vi "HeartBeatDetectOffline2Valsalva.vi"() -> ()   [LabVIEW 2014, in "Phonocardiography.lvlib"]
uses:
  Phonocardiography.lvlib
  <vilib>/Waveform/WDTOps.llb/WDT Index Channel DBL.vi
  <vilib>/Waveform/WDTOps.llb/WDT Get Waveform Time Array DBL.vi
  <vilib>/gmath/NI_Gmath.lvlib
  <vilib>/Analysis/NI_AALBase.lvlib
panel:
  in  "Exhale Length [s]":dbl=20.0
  out "RR intervals Spectra":T1(graph)={"Power Spectrum FFT {X} Frequency"=[0.0, 0.025494335748261657, 0.050988671496523315, 0.07648300724478498, 0.10197734299304663, 0.1274716787413083, 0.15296601448956995, 0.1784603502378316, 0.20395468598609326, 0.2294490217343549, 0.2549433574826166, 0.28043769323087825, 0.3059320289791399, 0.33142636472740156, 0.3569207004756632, 0.38241503622392486, 0.4079093719721865, 0.4334037077204482, 0.4588980434687098, 0.4843923792169715, 0.5098867149652332, 0.5353810507134948, 0.5608753864617565, 0.5863697222100182, 0.6118640579582798, 0.6373583937065415, 0.6628527294548031, 0.6883470652030648, 0.7138414009513264, 0.7393357366995881, 0.7648300724478497, 0.7903244081961114, 0.815818743944373, 0.8413130796926347, 0.8668074154408963, 0.892301751189158, 0.9177960869374197, 0.9432904226856813, 0.968784758433943, 0.9942790941822046, 1.0197734299304664, 1.045267765678728, 1.0707621014269897, 1.0962564371752512, 1.121750772923513, 1.1472451086717745, 1.1727394444200363, 1.1982337801682978, 1.2237281159165596, 1.2492224516648212, 1.274716787413083, 1.3002111231613445, 1.3257054589096062, 1.3511997946578678, 1.3766941304061295, 1.402188466154391, 1.4276828019026528, 1.4531771376509144, 1.4786714733991762], "Power Spectrum FFT {X}"=[6.194748647147158e-24, 9229.548494920025, 1188.4920860052935, 947.8842969704942, 178.63197208555547, 71.46762690308067, 205.39345276047945, 144.27075798793635, 81.13456035019907, 14.233100403863002, 70.63257760443297, 81.86763326737034, 31.359253750538112, 38.78063411373954, 63.199253406710866, 37.96608881281612, 1.8581095317295782, 7.247275056105265, 3.888477791210256, 19.078038441682054, 43.408583710979855, 31.794851712590184, 23.507910464090752, 3.0603332942735766, 9.734464709591705, 7.800318484915491, 22.688612828789623, 46.34799950953906, 30.540582735785772, 17.053473818925937, 5.267363301568957, 26.95792599083291, 10.575021658989519, 26.04160962099042, 119.40238100275175, 39.36493765074656, 47.92746655778191, 26.235986845520635, 199.6106688709268, 677.5407288058668, 356.86867414086265, 1572.0901514152968, 2451.586051527142, 477.6196783700457, 610.6344556635514, 1181.337476994924, 128.33756322878241, 687.9177159050421, 1078.297501063014, 1180.2511971323859, 289.91558302839945, 85.34770217036714, 78.25445989986403, 7.873565805919232, 82.9457034917068, 122.5040965317584, 14.428981027927678, 14.60917219116577, 2.0649497624039586]}
  in  "Remove\nEctopic Beats":bool=TRUE
  out "pNN50 [%]":dbl=10.344827586206897 format="%.1f"
  out "rMSSD  [ms] 2":dbl=56.69079988743271
  out "sdRR [ms]":dbl=155.73913956064249
  out "Mean RR [ms]":dbl=679.0314769975785 format="%_1f"
  out "Mean heart rate [BPM]":dbl=88.36114676936246 format="%#.1g"
  in  "Negate":bool
  out "Heart rate":T2(graph)=[{"X [s]"=[0.9536507936507932, 1.7804988662131511, 2.524807256235827, 3.2744671201814044, 4.085170068027209, 4.935691609977322, 5.717823129251698, 6.664217687074827, 7.49442176870748, 8.24662131519274, 8.931065759637184, 9.6128798185941, 10.405986394557818, 11.348027210884348, 12.258866213151922, 13.136780045351468, 13.961088435374144, 14.727165532879813, 15.434376417233553, 16.08961451247165, 16.721904761904756, 17.338321995464845, 17.933514739229018, 18.513469387755094, 19.077641723356003, 19.63292517006802, 20.182403628117907, 20.724172335600898, 21.26467120181405, 21.80018140589568, 22.325532879818585, 22.852698412698402, 23.38702947845804, 23.93859410430838, 24.48843537414965, 25.032743764172324, 25.566167800453503, 26.094965986394545, 26.626666666666654, 27.148843537414955, 27.667120181405885, 28.183219954648514, 28.69315192743763, 29.19600907029477, 29.70113378684806, 30.20426303854874, 30.718911564625838, 31.25142857142856, 31.85287981859409, 32.489795918367335, 33.11401360544216, 33.734331065759626, 34.587845804988646, 35.485986394557806, 36.427664399092954, 37.37106575963717, 38.321088435374136, 39.26984126984125, 40.178049886621295], "Heart Rate [BPM]"=[71.55993076590225, 72.56472136902153, 80.61174750182794, 80.03629764065343, 74.00984560304319, 70.54495041057912, 76.71344079786621, 63.39850488786662, 72.27138643067849, 79.76606776799711, 87.66233766233783, 88.0005321271783, 75.65187557182081, 63.69150779896015, 65.87333200557657, 68.34383717326173, 72.78829225352112, 78.32109874496807, 84.84032320123139, 91.56976744186045, 94.89312867594295, 97.33666862860537, 100.80768058518736, 103.45636534250875, 106.35048231511234, 108.05292388108468, 109.19445361505448, 110.74836765444552, 111.00855848296688, 112.04268292682941, 114.20925414364623, 113.81624225739887, 112.28993379731786, 108.78145041933905, 109.12240184757502, 110.2316280619899, 112.48087060023806, 113.4648370497429, 112.84544524053209, 114.90359562271999, 115.76828841442064, 116.25659050966627, 117.6627534685167, 119.31818181818207, 118.78254623810332, 119.25365062195846, 116.58442016214268, 112.67245784363834, 99.75870909365125, 94.20393050412952, 96.12031386225006, 96.72466734902676, 70.29755579171136, 66.80468592203607, 63.716047004430656, 63.599653879434875, 63.15638724460529, 63.240917782027125, 66.06411664835723]}, {"X [s]"=array[450560 elements], "Heart Rate [BPM]"=array[450560 elements]}]
  out "Heart beats":cluster{"Peaks X":dbl[], "Peaks Y":dbl[]}[](graph)=[{"Peaks X"=array[450560 elements], "Peaks Y"=array[450560 elements]}, {"Peaks X"=[0.11519274376417228, 0.9536507936507932, 1.7804988662131511, 2.524807256235827, 3.2744671201814044, 4.085170068027209, 4.935691609977322, 5.717823129251698, 6.664217687074827, 7.49442176870748, 8.24662131519274, 8.931065759637184, 9.6128798185941, 10.405986394557818, 11.348027210884348, 12.258866213151922, 13.136780045351468, 13.961088435374144, 14.727165532879813, 15.434376417233553, 16.08961451247165, 16.721904761904756, 17.338321995464845, 17.933514739229018, 18.513469387755094, 19.077641723356003, 19.63292517006802, 20.182403628117907, 20.724172335600898, 21.26467120181405, 21.80018140589568, 22.325532879818585, 22.852698412698402, 23.38702947845804, 23.93859410430838, 24.48843537414965, 25.032743764172324, 25.566167800453503, 26.094965986394545, 26.626666666666654, 27.148843537414955, 27.667120181405885, 28.183219954648514, 28.69315192743763, 29.19600907029477, 29.70113378684806, 30.20426303854874, 30.718911564625838, 31.25142857142856, 31.85287981859409, 32.489795918367335, 33.11401360544216, 33.734331065759626, 34.587845804988646, 35.485986394557806, 36.427664399092954, 37.37106575963717, 38.321088435374136, 39.26984126984125, 40.178049886621295], "Peaks Y"=[0.26409912109375, 0.216064453125, 0.231689453125, 0.2972412109375, 0.2186279296875, 0.310516357421875, 0.252410888671875, 0.3045654296875, 0.187164306640625, 0.24078369140625, 0.215057373046875, 0.3526611328125, 0.2615966796875, 0.229461669921875, 0.192779541015625, 0.189361572265625, 0.17205810546875, 0.186737060546875, 0.212005615234375, 0.185272216796875, 0.16400146484375, 0.175933837890625, 0.1873779296875, 0.1800537109375, 0.20709228515625, 0.20452880859375, 0.2001953125, 0.218231201171875, 0.222015380859375, 0.217681884765625, 0.201202392578125, 0.212066650390625, 0.219879150390625, 0.2449951171875, 0.2816162109375, 0.262664794921875, 0.234039306640625, 0.287567138671875, 0.267730712890625, 0.258544921875, 0.271209716796875, 0.25408935546875, 0.272186279296875, 0.230987548828125, 0.265380859375, 0.269317626953125, 0.267486572265625, 0.289703369140625, 0.216644287109375, 0.20257568359375, 0.270477294921875, 0.246978759765625, 0.403839111328125, 0.436309814453125, 0.427947998046875, 0.40887451171875, 0.40252685546875, 0.448974609375, 0.42376708984375, 0.371551513671875]}]
  in  "Max time to peak\nfrom threshold (ms)":dbl=150.0
  in  "Threshold mult 2":dbl=0.35 min=-1.0 max=1.0 step=0.05
  in  "Min time between\nbeats (ms)":dbl=400.0
  in  "width (threshold) 2":i32=3
  in  "File Path Control":path=path "C:/Users/Tamas/Documents/Projektek/Magzati szívhang/Felvételek cikkhez/valsalva5.wav"
  in  "Init length [s]":dbl=10.0
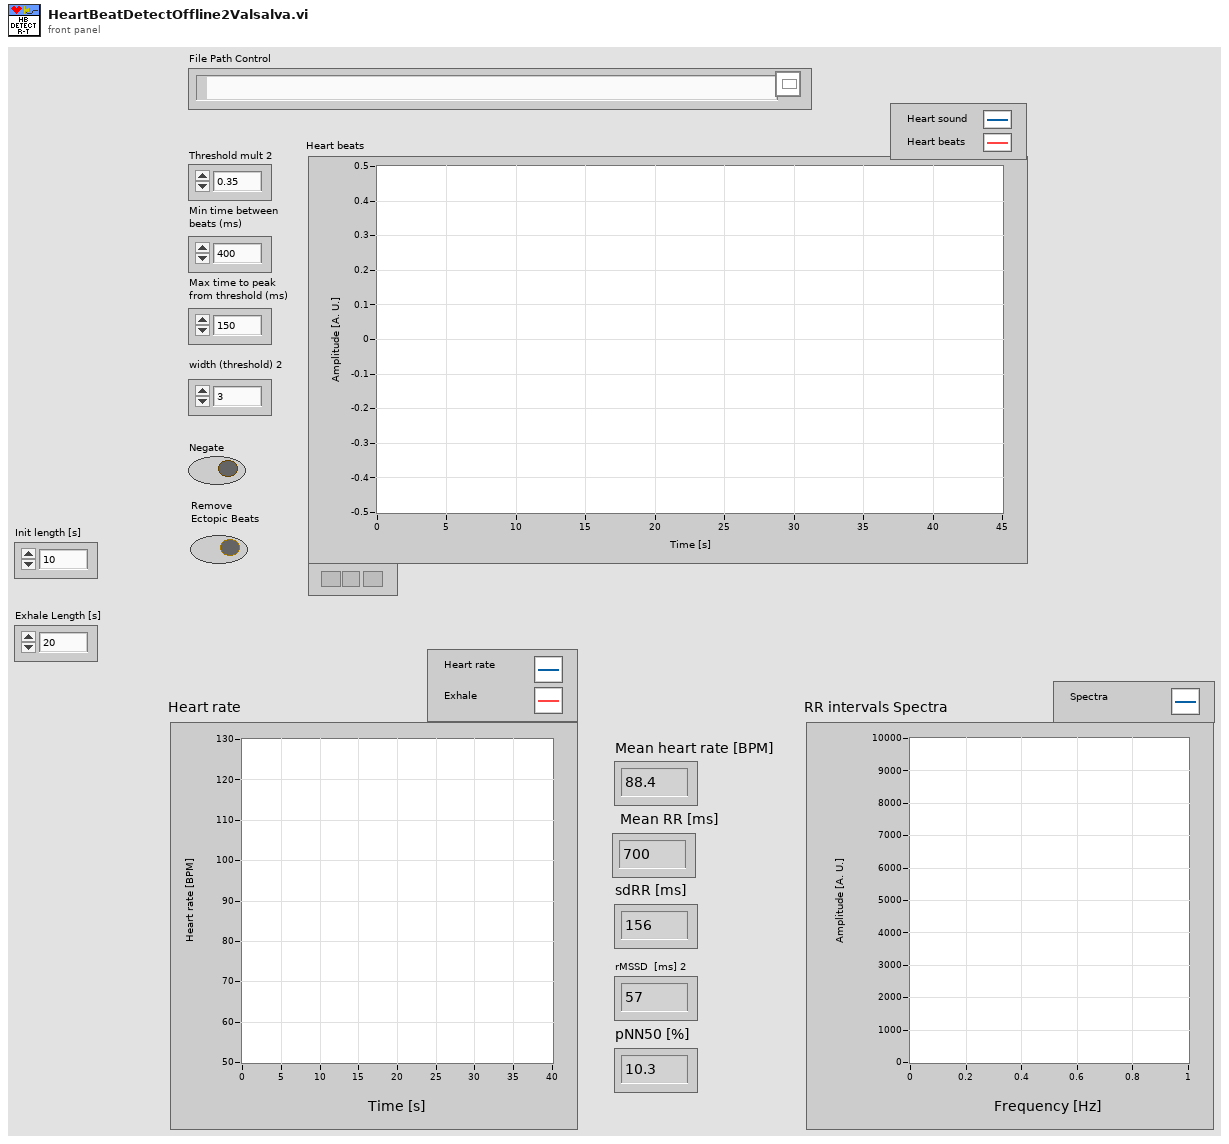
[diagram p1: front panel]
types:
  T1 = cluster{"Power Spectrum FFT {X} Frequency":dbl[], "Power Spectrum FFT {X}":dbl[]}
  T2 = cluster{"X [s]":dbl[], "Heart Rate [BPM]":dbl[]}[]
  T3 = typedef "LVCursorListTypeDef.ctl" = cluster{"Name":string, "Color":u32, "Style":u8, "Point Style":u8, "Name Visible":bool, "Allow Drag":bool, "Cursor Mode":u32, "Plot":i32, "Index":i32, "Position":cluster{"X":dbl, "Y":dbl}, "X Scale":u32, "Y Scale":u32, "Watch Plots":i32[], "Watch All Plots":bool, "Plot Area":i32, "Label Offset":cluster{"X":dbl, "Y":dbl}}[]
  T4 = cluster{"Name":string, "Color":u32, "Style":u8, "Point Style":u8, "Name Visible":bool, "Allow Drag":bool, "Cursor Mode":u32, "Plot":i32, "Index":i32, "Position":cluster{"X":dbl, "Y":dbl}, "X Scale":u32, "Y Scale":u32, "Watch Plots":i32[], "Watch All Plots":bool, "Plot Area":i32, "Label Offset":cluster{"X":dbl, "Y":dbl}}
  T5 = cluster{"Name":string, "Color":u32, "Style":u8, "Point Style":u8, "Name Visible":bool, "Allow Drag":bool, "Cursor Mode":u32, "Plot":i32, "Index":i32, "Position":cluster{"X":dbl, "Y":dbl}, "X Scale":u32, "Y Scale":u32, "Watch Plots":i32[], "Watch All Plots":bool, "Plot Area":i32, "Label Offset":cluster{"X":dbl, "Y":dbl}}[]
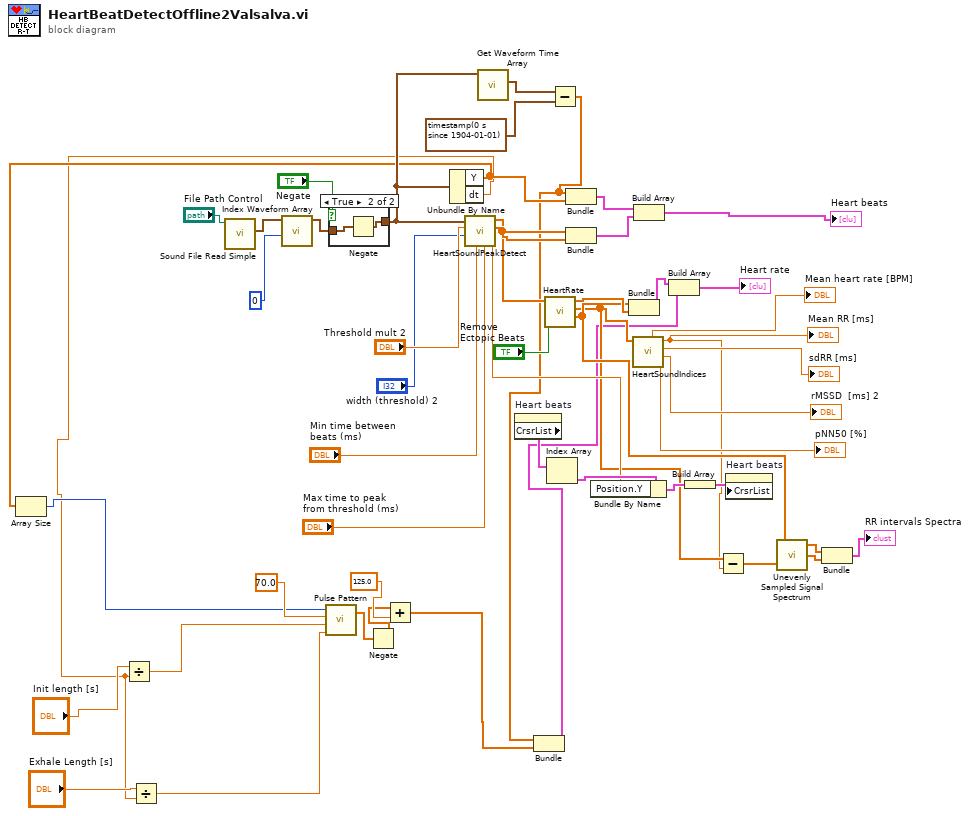
[diagram p0: block diagram]
diagram:
  n1 = call <vilib>:"Sound File Read Simple.vi"("path"="File Path Control") -> ("data"=w49:waveform(dbl)[])  [unwired: 7 in, 3 out]
  n2 = call-poly <vilib>:"Index Waveform Array.vi"("index"=0, "waveform array"=w49) -> ("waveform"=w30:waveform(dbl))  [unwired: 8 in, 1 out]
  n3 = case shown="True" "Negate" {
    tunnel: w30 -> [w52 w54]
    tunnel: [w52 w53] -> w29
    frame False {
    }
    frame True {
      n4 = Negate(x=w54) -> (-x=w53:waveform(dbl))
    }
  }
  n5 = Unbundle By Name(w29) -> ("Y"=w15:dbl[], "dt"=w6:dbl)
  n6 = Array Size(array=w15) -> (size(s)=w8:i32)
  n7 = Divide(x="Init length [s]", y=w6) -> (x/y=w4:dbl)
  n8 = Divide(x="Exhale Length [s]", y=w6) -> (x/y=w5:dbl)
  n9 = call <vilib>:"Pulse Pattern.vi"("width"=w5, "delay"=w4, "amplitude"=70.0, "samples"=w8) -> ("Pulse Pattern"=w2:dbl[])  [unwired: 1 out]
  n10 = Negate(x=w2) -> (-x=w1:dbl[])
  n11 = Add(x=w1, y=125.0 ("amplitude")) -> (x+y=w3:dbl[])
  n12 = call "HeartSoundPeakDetect.vi"("Max time to peak\nfrom threshold (ms)"="Max time to peak\nfrom threshold (ms)", "Min time between\nbeats (ms)"="Min time between\nbeats (ms)", "width (threshold)"="width (threshold) 2", "Threshold multiplier"="Threshold mult 2", "Sound"=w29) -> ("Threshold"=w31:dbl, "Peaks Y"=w43:dbl[], "Peaks X"=w40:dbl[])  [unwired: 4 in]
  n13 = call-poly <vilib>:"Get Waveform Time Array.vi"("waveform in"=w29) -> ("X array"=w38:timestamp[])  [unwired: 9 in, 1 out]
  n14 = property on="Heart beats" class="XYGraph (strict)"() -> ("CrsrList"=w33:T3)  [unwired: 2 in, 2 out]
  n15 = call "HeartRate.vi"("Remove Ectopic?"="Remove\nEctopic Beats", "Peaks X in"=w40) -> ("X [s]"=w22:dbl[], "RR intervals [ms]"=w17:dbl[], "Heart Rate [BPM]"=w39:dbl[])  [unwired: 7 in]
  n16 = Index Array(array=w33) -> (element=w35:T4)  [unwired: 1 in]
  n17 = Subtract(x=w38, y=timestamp(0 s since 1904-01-01) ("Xo")) -> (x-y=w14:dbl[])
  n18 = Bundle(w14, w3) -> (w12:cluster{dbl[], dbl[]})  [unwired: 1 in]
  n19 = Bundle(w14, "Y"=w15) -> (w42:cluster{dbl[], "Y":dbl[]})  [unwired: 1 in]
  n20 = Bundle("Peaks X"=w40, "Peaks Y"=w43) -> (w41:cluster{"Peaks X":dbl[], "Peaks Y":dbl[]})  [unwired: 1 in]
  n21 = Bundle By Name(cluster=w35, "Position.Y"=w31) -> (w34:T4)
  n22 = Bundle("X [s]"=w22, "Heart Rate [BPM]"=w39) -> (w13:cluster{"X [s]":dbl[], "Heart Rate [BPM]":dbl[]})  [unwired: 1 in]
  n23 = call "HeartSoundIndices.vi"("RR intervals [ms]"=w17) -> ("pNN50 [%]"=→"pNN50 [%]":dbl, "rMSSD  [ms]"=→"rMSSD  [ms] 2":dbl, "sdRR [ms]"=→"sdRR [ms]":dbl, "Mean RR [ms]"=w16:dbl, "Mean heart rate [BPM]"=→"Mean heart rate [BPM]":dbl)  [unwired: 6 in]
  "Mean RR [ms]" <- w16
  n24 = Build Array(w42, w41) -> (→"Heart beats":cluster{"Peaks X":dbl[], "Peaks Y":dbl[]}[])
  n25 = Build Array(w13, w12) -> (→"Heart rate":T2)
  n26 = Build Array(w34) -> (w32:T5)
  n27 = Subtract(x=w17, y=w16) -> (x-y=w18:dbl[])
  n28 = property on="Heart beats" class="XYGraph (strict)"("CrsrList"=w32) -> ()  [unwired: 2 in, 2 out]
  n29 = call <vilib>:"Unevenly Sampled Signal Spectrum.vi"("XTime"=w22, "X"=w18) -> ("Power Spectrum FFT {X} Frequency"=w21:dbl[], "Power Spectrum FFT {X}"=w20:dbl[])  [unwired: 1 out]
  n30 = Bundle("Power Spectrum FFT {X} Frequency"=w21, "Power Spectrum FFT {X}"=w20) -> (→"RR intervals Spectra":T1)  [unwired: 1 in]
